vi "1D history all datatypes.vi"   [LabVIEW 2021, in "Ring Buffer Strict Accessor Unit Tests.lvlib"] (continued)
  d3cdd860-2221-4504-b2d7-d7ebb0f0ee59.vi/38752bf6-7fea-4fd6-9295-87f253133584.vi/19bdd28a-0674-4be3-87bb-ec701e431d75.vi/2fb7b479-974d-4a18-8674-c4c8d9dc9a89.vi
  d3cdd860-2221-4504-b2d7-d7ebb0f0ee59.vi/38752bf6-7fea-4fd6-9295-87f253133584.vi/19bdd28a-0674-4be3-87bb-ec701e431d75.vi/faac7175-5814-4bb6-a961-a8db1f460653.vi
  d3cdd860-2221-4504-b2d7-d7ebb0f0ee59.vi/38752bf6-7fea-4fd6-9295-87f253133584.vi/19bdd28a-0674-4be3-87bb-ec701e431d75.vi/b6af2a6f-71a4-4cfe-837f-b196861458b0.vi
  ecb8fbaa-c9af-4774-8849-7f352d3a9ee1.vi/8499afdd-f86a-4785-a8f1-e7a09133571a.vi/f2df9050-0eef-46c6-aff6-3ce3a8893ea5.vi/63c583a5-c20f-4aba-9c90-661423dee4c4.vi
  ecb8fbaa-c9af-4774-8849-7f352d3a9ee1.vi/8499afdd-f86a-4785-a8f1-e7a09133571a.vi/f2df9050-0eef-46c6-aff6-3ce3a8893ea5.vi/52385341-3d9c-45d2-aff5-e082a4793eb1.vi
  ecb8fbaa-c9af-4774-8849-7f352d3a9ee1.vi/8499afdd-f86a-4785-a8f1-e7a09133571a.vi/f2df9050-0eef-46c6-aff6-3ce3a8893ea5.vi/37f29efa-f142-46b1-a185-f0098a95fbb6.vi
  ecb8fbaa-c9af-4774-8849-7f352d3a9ee1.vi/8499afdd-f86a-4785-a8f1-e7a09133571a.vi/f2df9050-0eef-46c6-aff6-3ce3a8893ea5.vi/84b3d231-9afe-4b6e-afae-e0be43a31e4e.vi
  ecb8fbaa-c9af-4774-8849-7f352d3a9ee1.vi/8499afdd-f86a-4785-a8f1-e7a09133571a.vi/f2df9050-0eef-46c6-aff6-3ce3a8893ea5.vi/c726271c-fc36-4bb7-8553-8945ec40c1cd.vi
  ecb8fbaa-c9af-4774-8849-7f352d3a9ee1.vi/8499afdd-f86a-4785-a8f1-e7a09133571a.vi/f2df9050-0eef-46c6-aff6-3ce3a8893ea5.vi/a7b1d944-dc88-46f5-9d3e-305d46bbe1f6.vi
  ecb8fbaa-c9af-4774-8849-7f352d3a9ee1.vi/8499afdd-f86a-4785-a8f1-e7a09133571a.vi/f2df9050-0eef-46c6-aff6-3ce3a8893ea5.vi/8abc4a6e-a1d2-4e85-879b-517e0ab55733.vi
  ecb8fbaa-c9af-4774-8849-7f352d3a9ee1.vi/8499afdd-f86a-4785-a8f1-e7a09133571a.vi/f2df9050-0eef-46c6-aff6-3ce3a8893ea5.vi/bd347357-b475-4a03-9ac5-3b85ef11aecc.vi
  ecb8fbaa-c9af-4774-8849-7f352d3a9ee1.vi/8499afdd-f86a-4785-a8f1-e7a09133571a.vi/f2df9050-0eef-46c6-aff6-3ce3a8893ea5.vi/391b36e9-a702-45e4-9499-3914f8833a58.vi
  ecb8fbaa-c9af-4774-8849-7f352d3a9ee1.vi/8499afdd-f86a-4785-a8f1-e7a09133571a.vi/f2df9050-0eef-46c6-aff6-3ce3a8893ea5.vi/44155b33-c915-49ce-9e44-a66693aa70dd.vi
  ecb8fbaa-c9af-4774-8849-7f352d3a9ee1.vi/8499afdd-f86a-4785-a8f1-e7a09133571a.vi/f2df9050-0eef-46c6-aff6-3ce3a8893ea5.vi/36977d53-dbe0-4dbc-b2ac-3dea4345b868.vi
  ecb8fbaa-c9af-4774-8849-7f352d3a9ee1.vi/38752bf6-7fea-4fd6-9295-87f253133584.vi/17d75e1a-130a-47e0-8f2c-6c7d90b8ca77.vi/bbb64351-fa28-4ac1-b583-44e271193ecd.vi
  ecb8fbaa-c9af-4774-8849-7f352d3a9ee1.vi/38752bf6-7fea-4fd6-9295-87f253133584.vi/19bdd28a-0674-4be3-87bb-ec701e431d75.vi/81c66277-30bd-484c-9c7c-9646f36721bb.vi
  ecb8fbaa-c9af-4774-8849-7f352d3a9ee1.vi/38752bf6-7fea-4fd6-9295-87f253133584.vi/19bdd28a-0674-4be3-87bb-ec701e431d75.vi/7ca10173-70f1-4bfb-9c4b-948090662032.vi
  ecb8fbaa-c9af-4774-8849-7f352d3a9ee1.vi/38752bf6-7fea-4fd6-9295-87f253133584.vi/19bdd28a-0674-4be3-87bb-ec701e431d75.vi/ea4aced9-3494-4b3f-b998-02af6afbdac4.vi
  ecb8fbaa-c9af-4774-8849-7f352d3a9ee1.vi/38752bf6-7fea-4fd6-9295-87f253133584.vi/19bdd28a-0674-4be3-87bb-ec701e431d75.vi/022c581c-5349-49df-98f9-5a038829ee63.vi
  ecb8fbaa-c9af-4774-8849-7f352d3a9ee1.vi/38752bf6-7fea-4fd6-9295-87f253133584.vi/19bdd28a-0674-4be3-87bb-ec701e431d75.vi/ed40bcc8-bbaa-4b61-9e1a-b4b75cf21b06.vi
  ecb8fbaa-c9af-4774-8849-7f352d3a9ee1.vi/38752bf6-7fea-4fd6-9295-87f253133584.vi/19bdd28a-0674-4be3-87bb-ec701e431d75.vi/f4b703c2-aaab-40a0-b3da-b0c22dc82d50.vi
  ecb8fbaa-c9af-4774-8849-7f352d3a9ee1.vi/38752bf6-7fea-4fd6-9295-87f253133584.vi/19bdd28a-0674-4be3-87bb-ec701e431d75.vi/1efa054f-b143-4d96-9f7e-584a7c6fa7fd.vi
  ecb8fbaa-c9af-4774-8849-7f352d3a9ee1.vi/38752bf6-7fea-4fd6-9295-87f253133584.vi/19bdd28a-0674-4be3-87bb-ec701e431d75.vi/b7c29f3f-256a-4401-af9d-aa15374df391.vi
  ecb8fbaa-c9af-4774-8849-7f352d3a9ee1.vi/38752bf6-7fea-4fd6-9295-87f253133584.vi/19bdd28a-0674-4be3-87bb-ec701e431d75.vi/2fb7b479-974d-4a18-8674-c4c8d9dc9a89.vi
  ecb8fbaa-c9af-4774-8849-7f352d3a9ee1.vi/38752bf6-7fea-4fd6-9295-87f253133584.vi/19bdd28a-0674-4be3-87bb-ec701e431d75.vi/faac7175-5814-4bb6-a961-a8db1f460653.vi
  ecb8fbaa-c9af-4774-8849-7f352d3a9ee1.vi/38752bf6-7fea-4fd6-9295-87f253133584.vi/19bdd28a-0674-4be3-87bb-ec701e431d75.vi/b6af2a6f-71a4-4cfe-837f-b196861458b0.vi
  dba9704d-e78e-47f3-8626-fce484395582.vi/8499afdd-f86a-4785-a8f1-e7a09133571a.vi/f2df9050-0eef-46c6-aff6-3ce3a8893ea5.vi/63c583a5-c20f-4aba-9c90-661423dee4c4.vi
  dba9704d-e78e-47f3-8626-fce484395582.vi/8499afdd-f86a-4785-a8f1-e7a09133571a.vi/f2df9050-0eef-46c6-aff6-3ce3a8893ea5.vi/52385341-3d9c-45d2-aff5-e082a4793eb1.vi
  dba9704d-e78e-47f3-8626-fce484395582.vi/8499afdd-f86a-4785-a8f1-e7a09133571a.vi/f2df9050-0eef-46c6-aff6-3ce3a8893ea5.vi/37f29efa-f142-46b1-a185-f0098a95fbb6.vi
  dba9704d-e78e-47f3-8626-fce484395582.vi/8499afdd-f86a-4785-a8f1-e7a09133571a.vi/f2df9050-0eef-46c6-aff6-3ce3a8893ea5.vi/84b3d231-9afe-4b6e-afae-e0be43a31e4e.vi
  dba9704d-e78e-47f3-8626-fce484395582.vi/8499afdd-f86a-4785-a8f1-e7a09133571a.vi/f2df9050-0eef-46c6-aff6-3ce3a8893ea5.vi/c726271c-fc36-4bb7-8553-8945ec40c1cd.vi
  dba9704d-e78e-47f3-8626-fce484395582.vi/8499afdd-f86a-4785-a8f1-e7a09133571a.vi/f2df9050-0eef-46c6-aff6-3ce3a8893ea5.vi/a7b1d944-dc88-46f5-9d3e-305d46bbe1f6.vi
  dba9704d-e78e-47f3-8626-fce484395582.vi/8499afdd-f86a-4785-a8f1-e7a09133571a.vi/f2df9050-0eef-46c6-aff6-3ce3a8893ea5.vi/8abc4a6e-a1d2-4e85-879b-517e0ab55733.vi
  dba9704d-e78e-47f3-8626-fce484395582.vi/8499afdd-f86a-4785-a8f1-e7a09133571a.vi/f2df9050-0eef-46c6-aff6-3ce3a8893ea5.vi/bd347357-b475-4a03-9ac5-3b85ef11aecc.vi
  dba9704d-e78e-47f3-8626-fce484395582.vi/8499afdd-f86a-4785-a8f1-e7a09133571a.vi/f2df9050-0eef-46c6-aff6-3ce3a8893ea5.vi/391b36e9-a702-45e4-9499-3914f8833a58.vi
  dba9704d-e78e-47f3-8626-fce484395582.vi/8499afdd-f86a-4785-a8f1-e7a09133571a.vi/f2df9050-0eef-46c6-aff6-3ce3a8893ea5.vi/44155b33-c915-49ce-9e44-a66693aa70dd.vi
  dba9704d-e78e-47f3-8626-fce484395582.vi/8499afdd-f86a-4785-a8f1-e7a09133571a.vi/f2df9050-0eef-46c6-aff6-3ce3a8893ea5.vi/36977d53-dbe0-4dbc-b2ac-3dea4345b868.vi
  dba9704d-e78e-47f3-8626-fce484395582.vi/38752bf6-7fea-4fd6-9295-87f253133584.vi/17d75e1a-130a-47e0-8f2c-6c7d90b8ca77.vi/bbb64351-fa28-4ac1-b583-44e271193ecd.vi
  dba9704d-e78e-47f3-8626-fce484395582.vi/38752bf6-7fea-4fd6-9295-87f253133584.vi/19bdd28a-0674-4be3-87bb-ec701e431d75.vi/81c66277-30bd-484c-9c7c-9646f36721bb.vi
  dba9704d-e78e-47f3-8626-fce484395582.vi/38752bf6-7fea-4fd6-9295-87f253133584.vi/19bdd28a-0674-4be3-87bb-ec701e431d75.vi/7ca10173-70f1-4bfb-9c4b-948090662032.vi
  dba9704d-e78e-47f3-8626-fce484395582.vi/38752bf6-7fea-4fd6-9295-87f253133584.vi/19bdd28a-0674-4be3-87bb-ec701e431d75.vi/ea4aced9-3494-4b3f-b998-02af6afbdac4.vi
  dba9704d-e78e-47f3-8626-fce484395582.vi/38752bf6-7fea-4fd6-9295-87f253133584.vi/19bdd28a-0674-4be3-87bb-ec701e431d75.vi/022c581c-5349-49df-98f9-5a038829ee63.vi
  dba9704d-e78e-47f3-8626-fce484395582.vi/38752bf6-7fea-4fd6-9295-87f253133584.vi/19bdd28a-0674-4be3-87bb-ec701e431d75.vi/ed40bcc8-bbaa-4b61-9e1a-b4b75cf21b06.vi
  dba9704d-e78e-47f3-8626-fce484395582.vi/38752bf6-7fea-4fd6-9295-87f253133584.vi/19bdd28a-0674-4be3-87bb-ec701e431d75.vi/f4b703c2-aaab-40a0-b3da-b0c22dc82d50.vi
  dba9704d-e78e-47f3-8626-fce484395582.vi/38752bf6-7fea-4fd6-9295-87f253133584.vi/19bdd28a-0674-4be3-87bb-ec701e431d75.vi/1efa054f-b143-4d96-9f7e-584a7c6fa7fd.vi
  dba9704d-e78e-47f3-8626-fce484395582.vi/38752bf6-7fea-4fd6-9295-87f253133584.vi/19bdd28a-0674-4be3-87bb-ec701e431d75.vi/b7c29f3f-256a-4401-af9d-aa15374df391.vi
  dba9704d-e78e-47f3-8626-fce484395582.vi/38752bf6-7fea-4fd6-9295-87f253133584.vi/19bdd28a-0674-4be3-87bb-ec701e431d75.vi/2fb7b479-974d-4a18-8674-c4c8d9dc9a89.vi
  dba9704d-e78e-47f3-8626-fce484395582.vi/38752bf6-7fea-4fd6-9295-87f253133584.vi/19bdd28a-0674-4be3-87bb-ec701e431d75.vi/faac7175-5814-4bb6-a961-a8db1f460653.vi
  dba9704d-e78e-47f3-8626-fce484395582.vi/38752bf6-7fea-4fd6-9295-87f253133584.vi/19bdd28a-0674-4be3-87bb-ec701e431d75.vi/b6af2a6f-71a4-4cfe-837f-b196861458b0.vi
  112621f5-6873-4c6d-a91b-c9d1466c59a4.vi/8499afdd-f86a-4785-a8f1-e7a09133571a.vi/f2df9050-0eef-46c6-aff6-3ce3a8893ea5.vi/63c583a5-c20f-4aba-9c90-661423dee4c4.vi
  112621f5-6873-4c6d-a91b-c9d1466c59a4.vi/8499afdd-f86a-4785-a8f1-e7a09133571a.vi/f2df9050-0eef-46c6-aff6-3ce3a8893ea5.vi/52385341-3d9c-45d2-aff5-e082a4793eb1.vi
  112621f5-6873-4c6d-a91b-c9d1466c59a4.vi/8499afdd-f86a-4785-a8f1-e7a09133571a.vi/f2df9050-0eef-46c6-aff6-3ce3a8893ea5.vi/37f29efa-f142-46b1-a185-f0098a95fbb6.vi
  112621f5-6873-4c6d-a91b-c9d1466c59a4.vi/8499afdd-f86a-4785-a8f1-e7a09133571a.vi/f2df9050-0eef-46c6-aff6-3ce3a8893ea5.vi/84b3d231-9afe-4b6e-afae-e0be43a31e4e.vi
  112621f5-6873-4c6d-a91b-c9d1466c59a4.vi/8499afdd-f86a-4785-a8f1-e7a09133571a.vi/f2df9050-0eef-46c6-aff6-3ce3a8893ea5.vi/c726271c-fc36-4bb7-8553-8945ec40c1cd.vi
  112621f5-6873-4c6d-a91b-c9d1466c59a4.vi/8499afdd-f86a-4785-a8f1-e7a09133571a.vi/f2df9050-0eef-46c6-aff6-3ce3a8893ea5.vi/a7b1d944-dc88-46f5-9d3e-305d46bbe1f6.vi
  112621f5-6873-4c6d-a91b-c9d1466c59a4.vi/8499afdd-f86a-4785-a8f1-e7a09133571a.vi/f2df9050-0eef-46c6-aff6-3ce3a8893ea5.vi/8abc4a6e-a1d2-4e85-879b-517e0ab55733.vi
  112621f5-6873-4c6d-a91b-c9d1466c59a4.vi/8499afdd-f86a-4785-a8f1-e7a09133571a.vi/f2df9050-0eef-46c6-aff6-3ce3a8893ea5.vi/bd347357-b475-4a03-9ac5-3b85ef11aecc.vi
  112621f5-6873-4c6d-a91b-c9d1466c59a4.vi/8499afdd-f86a-4785-a8f1-e7a09133571a.vi/f2df9050-0eef-46c6-aff6-3ce3a8893ea5.vi/391b36e9-a702-45e4-9499-3914f8833a58.vi
  112621f5-6873-4c6d-a91b-c9d1466c59a4.vi/8499afdd-f86a-4785-a8f1-e7a09133571a.vi/f2df9050-0eef-46c6-aff6-3ce3a8893ea5.vi/44155b33-c915-49ce-9e44-a66693aa70dd.vi
  112621f5-6873-4c6d-a91b-c9d1466c59a4.vi/8499afdd-f86a-4785-a8f1-e7a09133571a.vi/f2df9050-0eef-46c6-aff6-3ce3a8893ea5.vi/36977d53-dbe0-4dbc-b2ac-3dea4345b868.vi
  112621f5-6873-4c6d-a91b-c9d1466c59a4.vi/38752bf6-7fea-4fd6-9295-87f253133584.vi/17d75e1a-130a-47e0-8f2c-6c7d90b8ca77.vi/bbb64351-fa28-4ac1-b583-44e271193ecd.vi
  112621f5-6873-4c6d-a91b-c9d1466c59a4.vi/38752bf6-7fea-4fd6-9295-87f253133584.vi/19bdd28a-0674-4be3-87bb-ec701e431d75.vi/81c66277-30bd-484c-9c7c-9646f36721bb.vi
  112621f5-6873-4c6d-a91b-c9d1466c59a4.vi/38752bf6-7fea-4fd6-9295-87f253133584.vi/19bdd28a-0674-4be3-87bb-ec701e431d75.vi/7ca10173-70f1-4bfb-9c4b-948090662032.vi
  112621f5-6873-4c6d-a91b-c9d1466c59a4.vi/38752bf6-7fea-4fd6-9295-87f253133584.vi/19bdd28a-0674-4be3-87bb-ec701e431d75.vi/ea4aced9-3494-4b3f-b998-02af6afbdac4.vi
  112621f5-6873-4c6d-a91b-c9d1466c59a4.vi/38752bf6-7fea-4fd6-9295-87f253133584.vi/19bdd28a-0674-4be3-87bb-ec701e431d75.vi/022c581c-5349-49df-98f9-5a038829ee63.vi
  112621f5-6873-4c6d-a91b-c9d1466c59a4.vi/38752bf6-7fea-4fd6-9295-87f253133584.vi/19bdd28a-0674-4be3-87bb-ec701e431d75.vi/ed40bcc8-bbaa-4b61-9e1a-b4b75cf21b06.vi
  112621f5-6873-4c6d-a91b-c9d1466c59a4.vi/38752bf6-7fea-4fd6-9295-87f253133584.vi/19bdd28a-0674-4be3-87bb-ec701e431d75.vi/f4b703c2-aaab-40a0-b3da-b0c22dc82d50.vi
  112621f5-6873-4c6d-a91b-c9d1466c59a4.vi/38752bf6-7fea-4fd6-9295-87f253133584.vi/19bdd28a-0674-4be3-87bb-ec701e431d75.vi/1efa054f-b143-4d96-9f7e-584a7c6fa7fd.vi
  112621f5-6873-4c6d-a91b-c9d1466c59a4.vi/38752bf6-7fea-4fd6-9295-87f253133584.vi/19bdd28a-0674-4be3-87bb-ec701e431d75.vi/b7c29f3f-256a-4401-af9d-aa15374df391.vi
  112621f5-6873-4c6d-a91b-c9d1466c59a4.vi/38752bf6-7fea-4fd6-9295-87f253133584.vi/19bdd28a-0674-4be3-87bb-ec701e431d75.vi/2fb7b479-974d-4a18-8674-c4c8d9dc9a89.vi
  112621f5-6873-4c6d-a91b-c9d1466c59a4.vi/38752bf6-7fea-4fd6-9295-87f253133584.vi/19bdd28a-0674-4be3-87bb-ec701e431d75.vi/faac7175-5814-4bb6-a961-a8db1f460653.vi
  112621f5-6873-4c6d-a91b-c9d1466c59a4.vi/38752bf6-7fea-4fd6-9295-87f253133584.vi/19bdd28a-0674-4be3-87bb-ec701e431d75.vi/b6af2a6f-71a4-4cfe-837f-b196861458b0.vi
  7b287e7a-98f1-404d-bc95-c25095b4fc31.vi/8499afdd-f86a-4785-a8f1-e7a09133571a.vi/f2df9050-0eef-46c6-aff6-3ce3a8893ea5.vi/63c583a5-c20f-4aba-9c90-661423dee4c4.vi
  7b287e7a-98f1-404d-bc95-c25095b4fc31.vi/8499afdd-f86a-4785-a8f1-e7a09133571a.vi/f2df9050-0eef-46c6-aff6-3ce3a8893ea5.vi/52385341-3d9c-45d2-aff5-e082a4793eb1.vi
  7b287e7a-98f1-404d-bc95-c25095b4fc31.vi/8499afdd-f86a-4785-a8f1-e7a09133571a.vi/f2df9050-0eef-46c6-aff6-3ce3a8893ea5.vi/37f29efa-f142-46b1-a185-f0098a95fbb6.vi
  7b287e7a-98f1-404d-bc95-c25095b4fc31.vi/8499afdd-f86a-4785-a8f1-e7a09133571a.vi/f2df9050-0eef-46c6-aff6-3ce3a8893ea5.vi/84b3d231-9afe-4b6e-afae-e0be43a31e4e.vi
  7b287e7a-98f1-404d-bc95-c25095b4fc31.vi/8499afdd-f86a-4785-a8f1-e7a09133571a.vi/f2df9050-0eef-46c6-aff6-3ce3a8893ea5.vi/c726271c-fc36-4bb7-8553-8945ec40c1cd.vi
  7b287e7a-98f1-404d-bc95-c25095b4fc31.vi/8499afdd-f86a-4785-a8f1-e7a09133571a.vi/f2df9050-0eef-46c6-aff6-3ce3a8893ea5.vi/a7b1d944-dc88-46f5-9d3e-305d46bbe1f6.vi
  7b287e7a-98f1-404d-bc95-c25095b4fc31.vi/8499afdd-f86a-4785-a8f1-e7a09133571a.vi/f2df9050-0eef-46c6-aff6-3ce3a8893ea5.vi/8abc4a6e-a1d2-4e85-879b-517e0ab55733.vi
  7b287e7a-98f1-404d-bc95-c25095b4fc31.vi/8499afdd-f86a-4785-a8f1-e7a09133571a.vi/f2df9050-0eef-46c6-aff6-3ce3a8893ea5.vi/bd347357-b475-4a03-9ac5-3b85ef11aecc.vi
  7b287e7a-98f1-404d-bc95-c25095b4fc31.vi/8499afdd-f86a-4785-a8f1-e7a09133571a.vi/f2df9050-0eef-46c6-aff6-3ce3a8893ea5.vi/391b36e9-a702-45e4-9499-3914f8833a58.vi
  7b287e7a-98f1-404d-bc95-c25095b4fc31.vi/8499afdd-f86a-4785-a8f1-e7a09133571a.vi/f2df9050-0eef-46c6-aff6-3ce3a8893ea5.vi/44155b33-c915-49ce-9e44-a66693aa70dd.vi
  7b287e7a-98f1-404d-bc95-c25095b4fc31.vi/8499afdd-f86a-4785-a8f1-e7a09133571a.vi/f2df9050-0eef-46c6-aff6-3ce3a8893ea5.vi/36977d53-dbe0-4dbc-b2ac-3dea4345b868.vi
  7b287e7a-98f1-404d-bc95-c25095b4fc31.vi/38752bf6-7fea-4fd6-9295-87f253133584.vi/17d75e1a-130a-47e0-8f2c-6c7d90b8ca77.vi/bbb64351-fa28-4ac1-b583-44e271193ecd.vi
  7b287e7a-98f1-404d-bc95-c25095b4fc31.vi/38752bf6-7fea-4fd6-9295-87f253133584.vi/19bdd28a-0674-4be3-87bb-ec701e431d75.vi/81c66277-30bd-484c-9c7c-9646f36721bb.vi
  7b287e7a-98f1-404d-bc95-c25095b4fc31.vi/38752bf6-7fea-4fd6-9295-87f253133584.vi/19bdd28a-0674-4be3-87bb-ec701e431d75.vi/7ca10173-70f1-4bfb-9c4b-948090662032.vi
  7b287e7a-98f1-404d-bc95-c25095b4fc31.vi/38752bf6-7fea-4fd6-9295-87f253133584.vi/19bdd28a-0674-4be3-87bb-ec701e431d75.vi/ea4aced9-3494-4b3f-b998-02af6afbdac4.vi
  7b287e7a-98f1-404d-bc95-c25095b4fc31.vi/38752bf6-7fea-4fd6-9295-87f253133584.vi/19bdd28a-0674-4be3-87bb-ec701e431d75.vi/022c581c-5349-49df-98f9-5a038829ee63.vi
  7b287e7a-98f1-404d-bc95-c25095b4fc31.vi/38752bf6-7fea-4fd6-9295-87f253133584.vi/19bdd28a-0674-4be3-87bb-ec701e431d75.vi/ed40bcc8-bbaa-4b61-9e1a-b4b75cf21b06.vi
  7b287e7a-98f1-404d-bc95-c25095b4fc31.vi/38752bf6-7fea-4fd6-9295-87f253133584.vi/19bdd28a-0674-4be3-87bb-ec701e431d75.vi/f4b703c2-aaab-40a0-b3da-b0c22dc82d50.vi
  7b287e7a-98f1-404d-bc95-c25095b4fc31.vi/38752bf6-7fea-4fd6-9295-87f253133584.vi/19bdd28a-0674-4be3-87bb-ec701e431d75.vi/1efa054f-b143-4d96-9f7e-584a7c6fa7fd.vi
  7b287e7a-98f1-404d-bc95-c25095b4fc31.vi/38752bf6-7fea-4fd6-9295-87f253133584.vi/19bdd28a-0674-4be3-87bb-ec701e431d75.vi/b7c29f3f-256a-4401-af9d-aa15374df391.vi
  7b287e7a-98f1-404d-bc95-c25095b4fc31.vi/38752bf6-7fea-4fd6-9295-87f253133584.vi/19bdd28a-0674-4be3-87bb-ec701e431d75.vi/2fb7b479-974d-4a18-8674-c4c8d9dc9a89.vi
  7b287e7a-98f1-404d-bc95-c25095b4fc31.vi/38752bf6-7fea-4fd6-9295-87f253133584.vi/19bdd28a-0674-4be3-87bb-ec701e431d75.vi/faac7175-5814-4bb6-a961-a8db1f460653.vi
  7b287e7a-98f1-404d-bc95-c25095b4fc31.vi/38752bf6-7fea-4fd6-9295-87f253133584.vi/19bdd28a-0674-4be3-87bb-ec701e431d75.vi/b6af2a6f-71a4-4cfe-837f-b196861458b0.vi
  fa233392-5b64-4c8c-836f-c43556db6967.vi/8499afdd-f86a-4785-a8f1-e7a09133571a.vi/f2df9050-0eef-46c6-aff6-3ce3a8893ea5.vi/63c583a5-c20f-4aba-9c90-661423dee4c4.vi
  fa233392-5b64-4c8c-836f-c43556db6967.vi/8499afdd-f86a-4785-a8f1-e7a09133571a.vi/f2df9050-0eef-46c6-aff6-3ce3a8893ea5.vi/52385341-3d9c-45d2-aff5-e082a4793eb1.vi
  fa233392-5b64-4c8c-836f-c43556db6967.vi/8499afdd-f86a-4785-a8f1-e7a09133571a.vi/f2df9050-0eef-46c6-aff6-3ce3a8893ea5.vi/37f29efa-f142-46b1-a185-f0098a95fbb6.vi
  fa233392-5b64-4c8c-836f-c43556db6967.vi/8499afdd-f86a-4785-a8f1-e7a09133571a.vi/f2df9050-0eef-46c6-aff6-3ce3a8893ea5.vi/84b3d231-9afe-4b6e-afae-e0be43a31e4e.vi
  fa233392-5b64-4c8c-836f-c43556db6967.vi/8499afdd-f86a-4785-a8f1-e7a09133571a.vi/f2df9050-0eef-46c6-aff6-3ce3a8893ea5.vi/c726271c-fc36-4bb7-8553-8945ec40c1cd.vi
  fa233392-5b64-4c8c-836f-c43556db6967.vi/8499afdd-f86a-4785-a8f1-e7a09133571a.vi/f2df9050-0eef-46c6-aff6-3ce3a8893ea5.vi/a7b1d944-dc88-46f5-9d3e-305d46bbe1f6.vi
  fa233392-5b64-4c8c-836f-c43556db6967.vi/8499afdd-f86a-4785-a8f1-e7a09133571a.vi/f2df9050-0eef-46c6-aff6-3ce3a8893ea5.vi/8abc4a6e-a1d2-4e85-879b-517e0ab55733.vi
  fa233392-5b64-4c8c-836f-c43556db6967.vi/8499afdd-f86a-4785-a8f1-e7a09133571a.vi/f2df9050-0eef-46c6-aff6-3ce3a8893ea5.vi/bd347357-b475-4a03-9ac5-3b85ef11aecc.vi
  fa233392-5b64-4c8c-836f-c43556db6967.vi/8499afdd-f86a-4785-a8f1-e7a09133571a.vi/f2df9050-0eef-46c6-aff6-3ce3a8893ea5.vi/391b36e9-a702-45e4-9499-3914f8833a58.vi
  fa233392-5b64-4c8c-836f-c43556db6967.vi/8499afdd-f86a-4785-a8f1-e7a09133571a.vi/f2df9050-0eef-46c6-aff6-3ce3a8893ea5.vi/44155b33-c915-49ce-9e44-a66693aa70dd.vi
  fa233392-5b64-4c8c-836f-c43556db6967.vi/8499afdd-f86a-4785-a8f1-e7a09133571a.vi/f2df9050-0eef-46c6-aff6-3ce3a8893ea5.vi/36977d53-dbe0-4dbc-b2ac-3dea4345b868.vi
  fa233392-5b64-4c8c-836f-c43556db6967.vi/38752bf6-7fea-4fd6-9295-87f253133584.vi/17d75e1a-130a-47e0-8f2c-6c7d90b8ca77.vi/bbb64351-fa28-4ac1-b583-44e271193ecd.vi
  fa233392-5b64-4c8c-836f-c43556db6967.vi/38752bf6-7fea-4fd6-9295-87f253133584.vi/19bdd28a-0674-4be3-87bb-ec701e431d75.vi/81c66277-30bd-484c-9c7c-9646f36721bb.vi
  fa233392-5b64-4c8c-836f-c43556db6967.vi/38752bf6-7fea-4fd6-9295-87f253133584.vi/19bdd28a-0674-4be3-87bb-ec701e431d75.vi/7ca10173-70f1-4bfb-9c4b-948090662032.vi
  fa233392-5b64-4c8c-836f-c43556db6967.vi/38752bf6-7fea-4fd6-9295-87f253133584.vi/19bdd28a-0674-4be3-87bb-ec701e431d75.vi/ea4aced9-3494-4b3f-b998-02af6afbdac4.vi
  fa233392-5b64-4c8c-836f-c43556db6967.vi/38752bf6-7fea-4fd6-9295-87f253133584.vi/19bdd28a-0674-4be3-87bb-ec701e431d75.vi/022c581c-5349-49df-98f9-5a038829ee63.vi
  fa233392-5b64-4c8c-836f-c43556db6967.vi/38752bf6-7fea-4fd6-9295-87f253133584.vi/19bdd28a-0674-4be3-87bb-ec701e431d75.vi/ed40bcc8-bbaa-4b61-9e1a-b4b75cf21b06.vi
  fa233392-5b64-4c8c-836f-c43556db6967.vi/38752bf6-7fea-4fd6-9295-87f253133584.vi/19bdd28a-0674-4be3-87bb-ec701e431d75.vi/f4b703c2-aaab-40a0-b3da-b0c22dc82d50.vi
  fa233392-5b64-4c8c-836f-c43556db6967.vi/38752bf6-7fea-4fd6-9295-87f253133584.vi/19bdd28a-0674-4be3-87bb-ec701e431d75.vi/1efa054f-b143-4d96-9f7e-584a7c6fa7fd.vi
  fa233392-5b64-4c8c-836f-c43556db6967.vi/38752bf6-7fea-4fd6-9295-87f253133584.vi/19bdd28a-0674-4be3-87bb-ec701e431d75.vi/b7c29f3f-256a-4401-af9d-aa15374df391.vi
  fa233392-5b64-4c8c-836f-c43556db6967.vi/38752bf6-7fea-4fd6-9295-87f253133584.vi/19bdd28a-0674-4be3-87bb-ec701e431d75.vi/2fb7b479-974d-4a18-8674-c4c8d9dc9a89.vi
  fa233392-5b64-4c8c-836f-c43556db6967.vi/38752bf6-7fea-4fd6-9295-87f253133584.vi/19bdd28a-0674-4be3-87bb-ec701e431d75.vi/faac7175-5814-4bb6-a961-a8db1f460653.vi
  fa233392-5b64-4c8c-836f-c43556db6967.vi/38752bf6-7fea-4fd6-9295-87f253133584.vi/19bdd28a-0674-4be3-87bb-ec701e431d75.vi/b6af2a6f-71a4-4cfe-837f-b196861458b0.vi
  6d70e3f0-6966-4327-968b-3c5b2aebe7d0.vi/8499afdd-f86a-4785-a8f1-e7a09133571a.vi/f2df9050-0eef-46c6-aff6-3ce3a8893ea5.vi/63c583a5-c20f-4aba-9c90-661423dee4c4.vi
  6d70e3f0-6966-4327-968b-3c5b2aebe7d0.vi/8499afdd-f86a-4785-a8f1-e7a09133571a.vi/f2df9050-0eef-46c6-aff6-3ce3a8893ea5.vi/52385341-3d9c-45d2-aff5-e082a4793eb1.vi
  6d70e3f0-6966-4327-968b-3c5b2aebe7d0.vi/8499afdd-f86a-4785-a8f1-e7a09133571a.vi/f2df9050-0eef-46c6-aff6-3ce3a8893ea5.vi/37f29efa-f142-46b1-a185-f0098a95fbb6.vi
  6d70e3f0-6966-4327-968b-3c5b2aebe7d0.vi/8499afdd-f86a-4785-a8f1-e7a09133571a.vi/f2df9050-0eef-46c6-aff6-3ce3a8893ea5.vi/84b3d231-9afe-4b6e-afae-e0be43a31e4e.vi
  6d70e3f0-6966-4327-968b-3c5b2aebe7d0.vi/8499afdd-f86a-4785-a8f1-e7a09133571a.vi/f2df9050-0eef-46c6-aff6-3ce3a8893ea5.vi/c726271c-fc36-4bb7-8553-8945ec40c1cd.vi
  6d70e3f0-6966-4327-968b-3c5b2aebe7d0.vi/8499afdd-f86a-4785-a8f1-e7a09133571a.vi/f2df9050-0eef-46c6-aff6-3ce3a8893ea5.vi/a7b1d944-dc88-46f5-9d3e-305d46bbe1f6.vi
  6d70e3f0-6966-4327-968b-3c5b2aebe7d0.vi/8499afdd-f86a-4785-a8f1-e7a09133571a.vi/f2df9050-0eef-46c6-aff6-3ce3a8893ea5.vi/8abc4a6e-a1d2-4e85-879b-517e0ab55733.vi
  6d70e3f0-6966-4327-968b-3c5b2aebe7d0.vi/8499afdd-f86a-4785-a8f1-e7a09133571a.vi/f2df9050-0eef-46c6-aff6-3ce3a8893ea5.vi/bd347357-b475-4a03-9ac5-3b85ef11aecc.vi
  6d70e3f0-6966-4327-968b-3c5b2aebe7d0.vi/8499afdd-f86a-4785-a8f1-e7a09133571a.vi/f2df9050-0eef-46c6-aff6-3ce3a8893ea5.vi/391b36e9-a702-45e4-9499-3914f8833a58.vi
  6d70e3f0-6966-4327-968b-3c5b2aebe7d0.vi/8499afdd-f86a-4785-a8f1-e7a09133571a.vi/f2df9050-0eef-46c6-aff6-3ce3a8893ea5.vi/44155b33-c915-49ce-9e44-a66693aa70dd.vi
  6d70e3f0-6966-4327-968b-3c5b2aebe7d0.vi/8499afdd-f86a-4785-a8f1-e7a09133571a.vi/f2df9050-0eef-46c6-aff6-3ce3a8893ea5.vi/36977d53-dbe0-4dbc-b2ac-3dea4345b868.vi
  6d70e3f0-6966-4327-968b-3c5b2aebe7d0.vi/38752bf6-7fea-4fd6-9295-87f253133584.vi/17d75e1a-130a-47e0-8f2c-6c7d90b8ca77.vi/bbb64351-fa28-4ac1-b583-44e271193ecd.vi
  6d70e3f0-6966-4327-968b-3c5b2aebe7d0.vi/38752bf6-7fea-4fd6-9295-87f253133584.vi/19bdd28a-0674-4be3-87bb-ec701e431d75.vi/81c66277-30bd-484c-9c7c-9646f36721bb.vi
  6d70e3f0-6966-4327-968b-3c5b2aebe7d0.vi/38752bf6-7fea-4fd6-9295-87f253133584.vi/19bdd28a-0674-4be3-87bb-ec701e431d75.vi/7ca10173-70f1-4bfb-9c4b-948090662032.vi
  6d70e3f0-6966-4327-968b-3c5b2aebe7d0.vi/38752bf6-7fea-4fd6-9295-87f253133584.vi/19bdd28a-0674-4be3-87bb-ec701e431d75.vi/ea4aced9-3494-4b3f-b998-02af6afbdac4.vi
  6d70e3f0-6966-4327-968b-3c5b2aebe7d0.vi/38752bf6-7fea-4fd6-9295-87f253133584.vi/19bdd28a-0674-4be3-87bb-ec701e431d75.vi/022c581c-5349-49df-98f9-5a038829ee63.vi
  6d70e3f0-6966-4327-968b-3c5b2aebe7d0.vi/38752bf6-7fea-4fd6-9295-87f253133584.vi/19bdd28a-0674-4be3-87bb-ec701e431d75.vi/ed40bcc8-bbaa-4b61-9e1a-b4b75cf21b06.vi
  6d70e3f0-6966-4327-968b-3c5b2aebe7d0.vi/38752bf6-7fea-4fd6-9295-87f253133584.vi/19bdd28a-0674-4be3-87bb-ec701e431d75.vi/f4b703c2-aaab-40a0-b3da-b0c22dc82d50.vi
  6d70e3f0-6966-4327-968b-3c5b2aebe7d0.vi/38752bf6-7fea-4fd6-9295-87f253133584.vi/19bdd28a-0674-4be3-87bb-ec701e431d75.vi/1efa054f-b143-4d96-9f7e-584a7c6fa7fd.vi
  6d70e3f0-6966-4327-968b-3c5b2aebe7d0.vi/38752bf6-7fea-4fd6-9295-87f253133584.vi/19bdd28a-0674-4be3-87bb-ec701e431d75.vi/b7c29f3f-256a-4401-af9d-aa15374df391.vi
  6d70e3f0-6966-4327-968b-3c5b2aebe7d0.vi/38752bf6-7fea-4fd6-9295-87f253133584.vi/19bdd28a-0674-4be3-87bb-ec701e431d75.vi/2fb7b479-974d-4a18-8674-c4c8d9dc9a89.vi
  6d70e3f0-6966-4327-968b-3c5b2aebe7d0.vi/38752bf6-7fea-4fd6-9295-87f253133584.vi/19bdd28a-0674-4be3-87bb-ec701e431d75.vi/faac7175-5814-4bb6-a961-a8db1f460653.vi
  6d70e3f0-6966-4327-968b-3c5b2aebe7d0.vi/38752bf6-7fea-4fd6-9295-87f253133584.vi/19bdd28a-0674-4be3-87bb-ec701e431d75.vi/b6af2a6f-71a4-4cfe-837f-b196861458b0.vi
  <userlib>/bjustice/Ring Buffer for Time Series Data/SubVIs/Enforce array size multiple timestamps.vi
  Source/API/New.vi
  <vilib>/Utility/error.llb/Error Cluster From Error Code.vi
  <vilib>/Utility/error.llb/Trim Whitespace.vi
  Source/API/Destroy.vi
  <vilib>/addons/_JKI Toolkits/Caraya/classes/Assert/Assert Not Error.vi
  <vilib>/addons/_JKI Toolkits/Caraya/classes/Assert/Assert True.vi
  <vilib>/addons/_JKI Toolkits/Caraya/classes/Assert/Assert.lvclass
  <vilib>/addons/_JKI Toolkits/Caraya/classes/Test/Test.lvclass
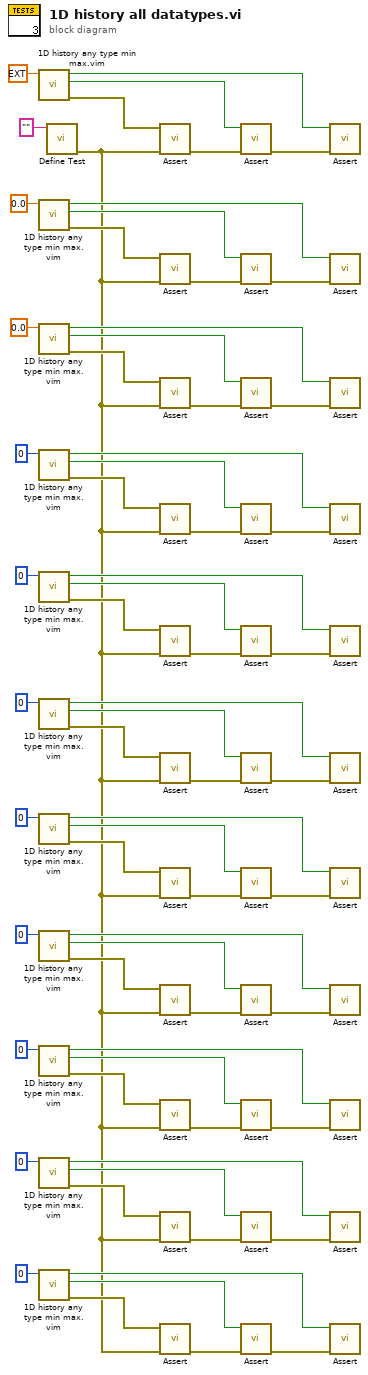
[diagram p0: block diagram]
diagram:
  n1 = call "1D history any type min max.vim"("Type"=ext 0.0 ("Numeric")) -> ("error out"=w66:errorcluster, "data equal?"=w64:bool, "timestamps equal?"=w65:bool)  [unwired: 8 in]
  n2 = call "1D history any type min max.vim"("Type"=0.0 ("Numeric")) -> ("error out"=w57:errorcluster, "data equal?"=w59:bool, "timestamps equal?"=w58:bool)  [unwired: 8 in]
  n3 = call "1D history any type min max.vim"("Type"=sgl 0.0 ("Numeric")) -> ("error out"=w54:errorcluster, "data equal?"=w52:bool, "timestamps equal?"=w53:bool)  [unwired: 8 in]
  n4 = call "1D history any type min max.vim"("Type"=i64 0 ("Numeric")) -> ("error out"=w45:errorcluster, "data equal?"=w47:bool, "timestamps equal?"=w46:bool)  [unwired: 8 in]
  n5 = call "1D history any type min max.vim"("Type"=0 ("Numeric")) -> ("error out"=w42:errorcluster, "data equal?"=w40:bool, "timestamps equal?"=w41:bool)  [unwired: 8 in]
  n6 = call "1D history any type min max.vim"("Type"=i16 0 ("Numeric")) -> ("error out"=w33:errorcluster, "data equal?"=w35:bool, "timestamps equal?"=w34:bool)  [unwired: 8 in]
  n7 = call "1D history any type min max.vim"("Type"=i8 0 ("Numeric")) -> ("error out"=w30:errorcluster, "data equal?"=w28:bool, "timestamps equal?"=w29:bool)  [unwired: 8 in]
  n8 = call "1D history any type min max.vim"("Type"=u64 0 ("Numeric")) -> ("error out"=w21:errorcluster, "data equal?"=w23:bool, "timestamps equal?"=w22:bool)  [unwired: 8 in]
  n9 = call "1D history any type min max.vim"("Type"=u32 0 ("Numeric")) -> ("error out"=w18:errorcluster, "data equal?"=w16:bool, "timestamps equal?"=w17:bool)  [unwired: 8 in]
  n10 = call "1D history any type min max.vim"("Type"=u16 0 ("Numeric")) -> ("error out"=w9:errorcluster, "data equal?"=w11:bool, "timestamps equal?"=w10:bool)  [unwired: 8 in]
  n11 = call "1D history any type min max.vim"("Type"=u8 0 ("Numeric")) -> ("error out"=w6:errorcluster, "data equal?"=w4:bool, "timestamps equal?"=w5:bool)  [unwired: 8 in]
  n12 = call <vilib>:"Define Test.vi"("Label (VI Title)"="") -> ("error out"=w1:errorcluster)  [unwired: 9 in, 1 out]
  n13 = call-poly <vilib>:"Assert.vi"("error in (no error)"=w1, "Not Error?"=w66) -> ("error out"=w63:errorcluster)  [unwired: 8 in, 1 out]
  n14 = call-poly <vilib>:"Assert.vi"("error in (no error)"=w1, "Not Error?"=w57) -> ("error out"=w60:errorcluster)  [unwired: 8 in, 1 out]
  n15 = call-poly <vilib>:"Assert.vi"("error in (no error)"=w1, "Not Error?"=w54) -> ("error out"=w51:errorcluster)  [unwired: 8 in, 1 out]
  n16 = call-poly <vilib>:"Assert.vi"("error in (no error)"=w1, "Not Error?"=w45) -> ("error out"=w48:errorcluster)  [unwired: 8 in, 1 out]
  n17 = call-poly <vilib>:"Assert.vi"("error in (no error)"=w1, "Not Error?"=w42) -> ("error out"=w39:errorcluster)  [unwired: 8 in, 1 out]
  n18 = call-poly <vilib>:"Assert.vi"("error in (no error)"=w1, "Not Error?"=w33) -> ("error out"=w36:errorcluster)  [unwired: 8 in, 1 out]
  n19 = call-poly <vilib>:"Assert.vi"("error in (no error)"=w1, "Not Error?"=w30) -> ("error out"=w27:errorcluster)  [unwired: 8 in, 1 out]
  n20 = call-poly <vilib>:"Assert.vi"("error in (no error)"=w1, "Not Error?"=w21) -> ("error out"=w24:errorcluster)  [unwired: 8 in, 1 out]
  n21 = call-poly <vilib>:"Assert.vi"("error in (no error)"=w1, "Not Error?"=w18) -> ("error out"=w15:errorcluster)  [unwired: 8 in, 1 out]
  n22 = call-poly <vilib>:"Assert.vi"("error in (no error)"=w1, "Not Error?"=w9) -> ("error out"=w12:errorcluster)  [unwired: 8 in, 1 out]
  n23 = call-poly <vilib>:"Assert.vi"("error in (no error)"=w1, "Not Error?"=w6) -> ("error out"=w3:errorcluster)  [unwired: 8 in, 1 out]
  n24 = call-poly <vilib>:"Assert.vi"("error in (no error)"=w63, "True?"=w64) -> ("error out"=w62:errorcluster)  [unwired: 8 in, 1 out]
  n25 = call-poly <vilib>:"Assert.vi"("error in (no error)"=w60, "True?"=w59) -> ("error out"=w61:errorcluster)  [unwired: 8 in, 1 out]
  n26 = call-poly <vilib>:"Assert.vi"("error in (no error)"=w51, "True?"=w52) -> ("error out"=w50:errorcluster)  [unwired: 8 in, 1 out]
  n27 = call-poly <vilib>:"Assert.vi"("error in (no error)"=w48, "True?"=w47) -> ("error out"=w49:errorcluster)  [unwired: 8 in, 1 out]
  n28 = call-poly <vilib>:"Assert.vi"("error in (no error)"=w39, "True?"=w40) -> ("error out"=w38:errorcluster)  [unwired: 8 in, 1 out]
  n29 = call-poly <vilib>:"Assert.vi"("error in (no error)"=w36, "True?"=w35) -> ("error out"=w37:errorcluster)  [unwired: 8 in, 1 out]
  n30 = call-poly <vilib>:"Assert.vi"("error in (no error)"=w27, "True?"=w28) -> ("error out"=w26:errorcluster)  [unwired: 8 in, 1 out]
  n31 = call-poly <vilib>:"Assert.vi"("error in (no error)"=w24, "True?"=w23) -> ("error out"=w25:errorcluster)  [unwired: 8 in, 1 out]
  n32 = call-poly <vilib>:"Assert.vi"("error in (no error)"=w15, "True?"=w16) -> ("error out"=w14:errorcluster)  [unwired: 8 in, 1 out]
  n33 = call-poly <vilib>:"Assert.vi"("error in (no error)"=w12, "True?"=w11) -> ("error out"=w13:errorcluster)  [unwired: 8 in, 1 out]
  n34 = call-poly <vilib>:"Assert.vi"("error in (no error)"=w3, "True?"=w4) -> ("error out"=w2:errorcluster)  [unwired: 8 in, 1 out]
  n35 = call-poly <vilib>:"Assert.vi"("error in (no error)"=w62, "True?"=w65) -> ()  [unwired: 8 in, 2 out]
  n36 = call-poly <vilib>:"Assert.vi"("error in (no error)"=w61, "True?"=w58) -> ()  [unwired: 8 in, 2 out]
  n37 = call-poly <vilib>:"Assert.vi"("error in (no error)"=w50, "True?"=w53) -> ()  [unwired: 8 in, 2 out]
  n38 = call-poly <vilib>:"Assert.vi"("error in (no error)"=w49, "True?"=w46) -> ()  [unwired: 8 in, 2 out]
  n39 = call-poly <vilib>:"Assert.vi"("error in (no error)"=w38, "True?"=w41) -> ()  [unwired: 8 in, 2 out]
  n40 = call-poly <vilib>:"Assert.vi"("error in (no error)"=w37, "True?"=w34) -> ()  [unwired: 8 in, 2 out]
  n41 = call-poly <vilib>:"Assert.vi"("error in (no error)"=w26, "True?"=w29) -> ()  [unwired: 8 in, 2 out]
  n42 = call-poly <vilib>:"Assert.vi"("error in (no error)"=w25, "True?"=w22) -> ()  [unwired: 8 in, 2 out]
  n43 = call-poly <vilib>:"Assert.vi"("error in (no error)"=w14, "True?"=w17) -> ()  [unwired: 8 in, 2 out]
  n44 = call-poly <vilib>:"Assert.vi"("error in (no error)"=w13, "True?"=w10) -> ()  [unwired: 8 in, 2 out]
  n45 = call-poly <vilib>:"Assert.vi"("error in (no error)"=w2, "True?"=w5) -> ()  [unwired: 8 in, 2 out]
